vi "45-1523-1 State Diagram.vi"() -> ()   [LabVIEW 2015]
uses:
  Cases.ctl
  <vilib>/DAQmx/read.llb/DAQmx Read (Analog DBL 1Chan 1Samp).vi
  <vilib>/DAQmx/write.llb/DAQmx Write (Digital Bool 1Line 1Point).vi
  <vilib>/DAQmx/miscellaneous.llb/DAQmx Fill In Error Info.vi
  <vilib>/ErrorRing/Error Ring.xnode
  <vilib>/LabVIEW Interface for Arduino/LabVIEW Interface for Arduino.lvlib
panel:
  out "Numeric 3":dbl
  out "Numeric 2":dbl
  in  "EXIT Button":bool
  out "Numeric":dbl
  in  "Tab Control":T1(tab)
  in  "START Button":bool
  out "Slide":u8(slide) scale=0.0..100.0
  out "Slide 2":u8(slide) scale=0.0..100.0
  out "Slide 3":u8(slide) scale=0.0..100.0
  out "Slide 4":u8(slide) scale=0.0..100.0
  in  "Restart Button":bool
  in  "OK Button":bool
  in  "OK Button 10":bool
  in  "OK Button 3":bool
  in  "OK Button 4":bool
  in  "Restart Button 2":bool
  in  "START Button 2":bool caption="START Button"
  in  "OK Button 5":bool
  in  "OK Button 6":bool
  in  "OK Button 7":bool
  in  "OK Button 8":bool
  out "Slide 5":u8(slide) scale=0.0..100.0
  in  "OK Button 9":bool
  in  "OK Button 11":bool
  in  "OK Button 12":bool
  # "45-1523-1 Functional Tester"
  # "Click \"START TEST\" To Begin Test"
  # "TESTING J15..."
  # "TESTING K2..."
  # "TESTING K3..."
  # "TESTING K4..."
  # "ALL TESTS PASSED!"
  # "CHECK HIGHLIGHTED CONNECTIONS"
  # "SWITCH K2 FAILED!"
  # "SWITCH K3 FAILED!"
  # "SWITCH K4 FAILED!"
  # "Test Failed"
  # "Verify Connections, then Click \"START\""
  # "Possible Locations of Failure:\n   - Switch K1\n   - S1 Jumper\n   - Q4\n   - U1\n   - Q5"
  # "CHECK HIGHLIGHTED CONNECTIONS"
  # "Power Fault to Board"
  # "CHECK HIGHLIGHTED CONNECTION"
  # "TESTING DUT Power..."
  # "Are All Three LEDs Lit?"
  # "Possible Causes of Failure:\n   - LEDs (Reversed or Faulty)\n   - U1\n   - Q2"
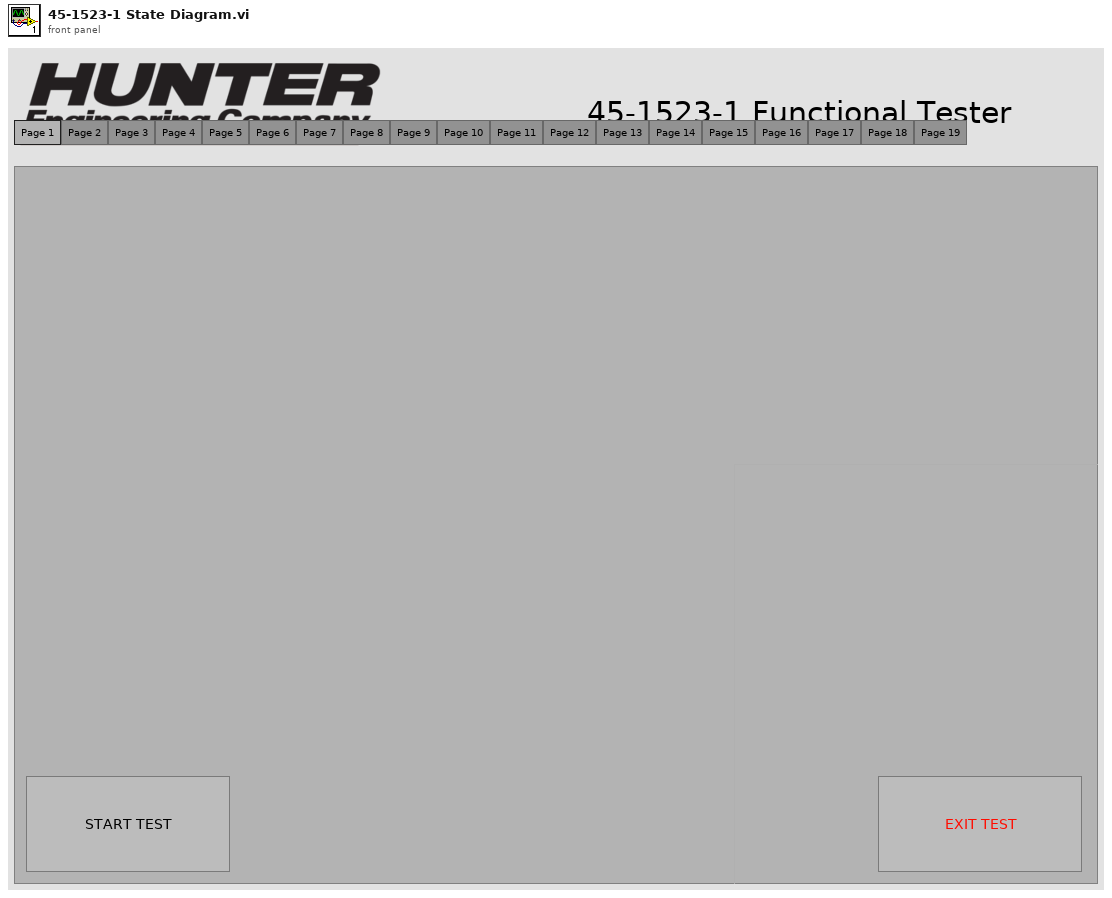
[diagram p1: front panel]
types:
  T1 = enum32{"Page 1", "Page 2", "Page 3", "Page 4", "Page 5", "Page 6", "Page 7", "Page 8", "Page 9", "Page 10", "Page 11", "Page 12", "Page 13", "Page 14", "Page 15", "Page 16", "Page 17", "Page 18", "Page 19"}
  T2 = typedef "Cases.ctl" = enum16{"Start", "Initalization", "J16 Test", "J15 Test", "J15 Error Page", "K2 Test", "K2 Error Page", "K3 Test", "K3 Error Page", "K4 Test", "K4 Error Page", "Test Complete", "Test Failed", "Error", "J15 Failed", "J16 Error", "J16 Failed", "K2 Failed", "LEDs Failed"}
  T3 = typedef "LabVIEW Interface for Arduino.lvlib/Arduino Resource.ctl" = cluster{"VISA resource":refnum<visa-resource-name>, "Board Type":T4, "Connection Type":enum8{"USB / Serial"}, "Bytes Per Packet (15)":u8}
  T4 = typedef "LabVIEW Interface for Arduino.lvlib/Board Type.ctl" = enum16{"Uno", "Dimuelanove w/Atmega 328", "Mega 2560"}
  T5 = enum8{"Enabled", "Disabled", "Disabled and Grayed Out"}
  T6 = enum32{"Page 1", "Page 2", "Page 3", "Page 4", "Page 5", "Page 6", "Page 7", "Page 8", "Page 9", "Page 10", "Page 11"}
  T7 = enum32{"Page 1", "Page 2", "Page 3", "Page 4", "Page 5", "Page 6", "Page 7", "Page 8", "Page 9", "Page 10", "Page 11", "Page 12"}
  T8 = enum32{"Page 1", "Page 2", "Page 3", "Page 4", "Page 5", "Page 6", "Page 7", "Page 8", "Page 9", "Page 10", "Page 11", "Page 12", "Page 13", "Page 14", "Page 15", "Page 16", "Page 17"}
  T9 = enum32{"Page 1", "Page 2", "Page 3", "Page 4", "Page 5", "Page 6", "Page 7", "Page 8", "Page 9", "Page 10", "Page 11", "Page 12", "Page 13", "Page 14", "Page 15", "Page 16", "Page 17", "Page 18"}
  T10 = enum32{"Page 1", "Page 2", "Page 3", "Page 4", "Page 5", "Page 6", "Page 7", "Page 8", "Page 9", "Page 10", "Page 11", "Page 12", "Page 13", "Page 14", "Page 15", "Page 16"}
  T11 = enum32{"Page 1", "Page 2", "Page 3", "Page 4", "Page 5", "Page 6", "Page 7", "Page 8", "Page 9", "Page 10", "Page 11", "Page 12", "Page 13"}
  T12 = enum32{"Page 1", "Page 2", "Page 3", "Page 4", "Page 5", "Page 6", "Page 7", "Page 8", "Page 9", "Page 10", "Page 11", "Page 12", "Page 13", "Page 14"}
  T13 = enum32{"Page 1", "Page 2", "Page 3", "Page 4", "Page 5", "Page 6", "Page 7", "Page 8", "Page 9", "Page 10", "Page 11", "Page 12", "Page 13", "Page 14", "Page 15"}
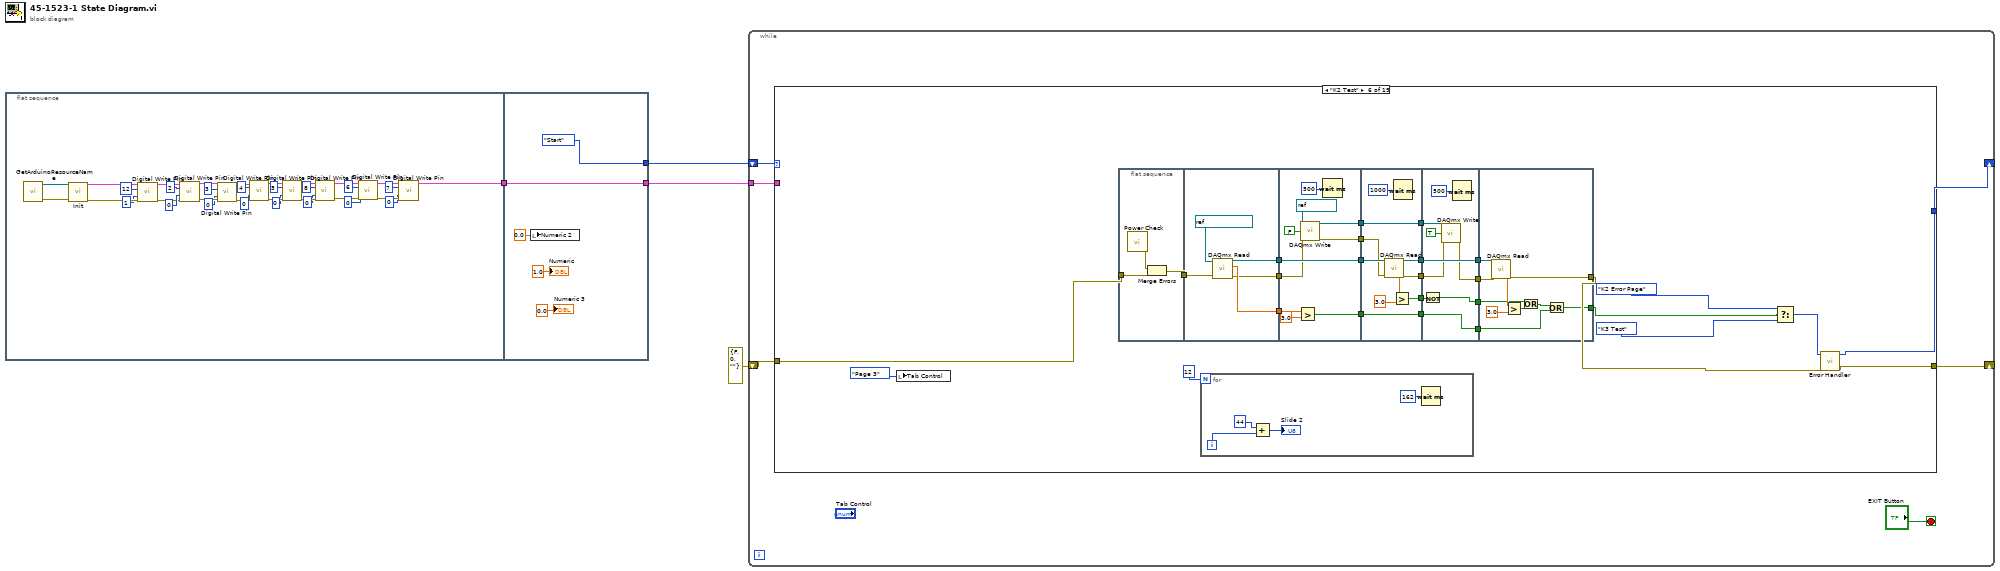
[diagram p0: block diagram]
diagram:
  n1 = flat-sequence {
    tunnel: [w11] -> w2
    tunnel: [Cases."Start" ("Enum")] -> w3
    tunnel: [w40] -> w1
    tunnel: w2 -> [w40]
    frame #0 {
      n2 = call "GetArduinoResourceName.vi"() -> ("error out"=w38:errorcluster, "VISA resource name"=w39:refnum<visa-resource-name>)  [unwired: 10 in]
      n3 = call <vilib>:"Init.vi"("VISA resource"=w39, "error in"=w38) -> ("Arduino Resource"=w10:T3, "error out"=w9:errorcluster)  [unwired: 16 in]
      n4 = call <vilib>:"Digital Write Pin.vi"("Arduino Resource"=w10, "Digital I/O Pin (0)"=u8 12, "Value (0)"=u8 1, "error in"=w9) -> ("Arduino Resource"=w7:T3, "error out"=w8:errorcluster)  [unwired: 10 in]
      n5 = call <vilib>:"Digital Write Pin.vi"("Arduino Resource"=w7, "Digital I/O Pin (0)"=u8 2, "Value (0)"=u8 0, "error in"=w8) -> ("Arduino Resource"=w37:T3, "error out"=w36:errorcluster)  [unwired: 10 in]
      n6 = call <vilib>:"Digital Write Pin.vi"("Arduino Resource"=w37, "Digital I/O Pin (0)"=u8 3, "Value (0)"=u8 0, "error in"=w36) -> ("Arduino Resource"=w35:T3, "error out"=w34:errorcluster)  [unwired: 10 in]
      n7 = call <vilib>:"Digital Write Pin.vi"("Arduino Resource"=w35, "Digital I/O Pin (0)"=u8 4, "Value (0)"=u8 0, "error in"=w34) -> ("Arduino Resource"=w33:T3, "error out"=w32:errorcluster)  [unwired: 10 in]
      n8 = call <vilib>:"Digital Write Pin.vi"("Arduino Resource"=w33, "Digital I/O Pin (0)"=u8 5, "Value (0)"=u8 0, "error in"=w32) -> ("Arduino Resource"=w31:T3, "error out"=w30:errorcluster)  [unwired: 10 in]
      n9 = call <vilib>:"Digital Write Pin.vi"("Arduino Resource"=w31, "Digital I/O Pin (0)"=u8 8, "Value (0)"=u8 0, "error in"=w30) -> ("Arduino Resource"=w19:T3, "error out"=w16:errorcluster)  [unwired: 10 in]
      n10 = call <vilib>:"Digital Write Pin.vi"("Arduino Resource"=w19, "Digital I/O Pin (0)"=u8 6, "Value (0)"=u8 0, "error in"=w16) -> ("Arduino Resource"=w14:T3, "error out"=w15:errorcluster)  [unwired: 10 in]
      n11 = call <vilib>:"Digital Write Pin.vi"("Arduino Resource"=w14, "Digital I/O Pin (0)"=u8 7, "Value (0)"=u8 0, "error in"=w15) -> ("Arduino Resource"=w11:T3)  [unwired: 10 in, 1 out]
    }
    frame #1 {
      n12 = local write "Numeric 2"(0.0 ("Numeric 2")) -> ()
      "Numeric" <- 1.0 ("Numeric")
      "Numeric 3" <- 0.0 ("Numeric 3")
    }
  }
  n13 = while {
    shift-right: [w49] -> _
    shift-left: w3 -> [w50]
    shift-right: [w47] -> _
    shift-left: errorcluster {"status"=FALSE, "code"=0, "source"=""} ("error out") -> [w46]
    tunnel: w1 -> [w45]
    stop <- "EXIT Button" stop-if-true
    n14 = case shown="\"K2 Test\"" w50 {
      tunnel: [w53 w78 w145 w206 w347 w383 w464 w479 w553 w575 w636 w645 w661 w680 w694 w706 w717 w727 w735] -> w49
      tunnel: [w55 w79 w144 w207 w348 w385 w465 w481 w556 w574 w635 w644 w660 w681 w693 w708 w719 w725 w737] -> w47
      tunnel: w46 -> [w51 w69 w142 w208 w342 w393 w466 w484 w555 w580 w634 w643 w653 w679 w692 w707 w720 w726 w736]
      tunnel: w45 -> [_ w68 w136 w177 w339 _ _ _ _ _ _ _ _ _ _ _ _ _ _]
      frame "Start" {
        n15 = property on="EXIT Button" class="Bool (strict)"("DisabledEnum"=T5."Enabled" ("Disabled")) -> ()  [unwired: 2 in, 2 out]
        n16 = while {
          stop <- w57 stop-if-true
          n17 = event shown="[0] \"START Button\", \"EXIT Button\": Value Change" {
            selector: _ -> [_]
            dyn-events: _ -> [_]
            timeout: _ -> [_]
            tunnel: ["START Button"] -> w57
            event "START Button", "EXIT Button": Value Change {
              n18 = event-data() -> ()  [unwired: 1 in, 6 out]
              n19 = local read "EXIT Button"() -> (w59:bool)
              n20 = case shown="False" w59 {
                tunnel: w59 -> [_ _]
                frame False {
                }
                frame True {
                  n21 = call "Shutdown VI.vi"() -> ()  [unwired: 12 in]
                }
              }
            }
          }
          n22 = local write "Tab Control"(T6."Page 1" ("Tab Control")) -> ()
        }
        n23 = call "Error Handler.vi"("error in (no error)"=w51, "Enum in"=Cases."Initalization") -> ("error out"=w55:errorcluster, "Enum out"=w53:T2)  [unwired: 8 in]
      }
      frame "Initalization", Default {
        n24 = local read "Numeric 2"() -> (w83:dbl)
        n25 = local write "Slide 5"(u8 0 ("Slide 5")) -> ()
        n26 = local write "Slide"(u8 22 ("Slide")) -> ()
        n27 = local write "Slide 2"(u8 40 ("Slide 2")) -> ()
        n28 = local write "Slide 3"(u8 52 ("Slide 3")) -> ()
        n29 = local write "Slide 4"(u8 67 ("Slide 4")) -> ()
        n30 = property on="EXIT Button" class="Bool (strict)"("DisabledEnum"=T5."Enabled" ("Disabled")) -> ()  [unwired: 2 in, 2 out]
        n31 = Equal?(x=2.0, y=w83) -> (x = y?=w82:bool)
        n32 = case shown="False" w82 {
          frame False {
          }
          frame True {
            "Numeric 2" <- 0.0 ("Numeric 2")
          }
        }
        n33 = flat-sequence {
          tunnel: [Cases."J16 Test" ("Enum")] -> w67
          tunnel: [w92] -> w65
          tunnel: w68 -> [w92]
          tunnel: w67 -> [w99]
          tunnel: [w99] -> w66
          tunnel: w65 -> [w98]
          tunnel: [w98] -> w64
          tunnel: w66 -> [w104]
          tunnel: [w104] -> w63
          tunnel: w64 -> [w103]
          tunnel: [w102] -> w61
          tunnel: w63 -> [w107]
          tunnel: [w107] -> w62
          tunnel: w61 -> [w106]
          tunnel: [w106] -> w60
          tunnel: w62 -> [w113]
          tunnel: [w114] -> w80
          tunnel: [w113] -> w77
          tunnel: w60 -> [w110]
          frame #0 {
            n34 = while {
              stop <- "START Button 2" stop-if-true
              n35 = local read "EXIT Button"() -> (w95:bool)
              n36 = case shown="False" w95 {
                frame False {
                }
                frame True {
                  n37 = call "Shutdown VI.vi"() -> ()  [unwired: 12 in]
                }
              }
            }
            n38 = local write "Tab Control"(T7."Page 12" ("Tab Control")) -> ()
          }
          frame #1 {
            n39 = Wait (ms)(milliseconds to wait=u32 1000) -> ()  [unwired: 1 out]
          }
          frame #2 {
            n40 = call <vilib>:"Digital Write Pin.vi"("Arduino Resource"=w103, "Digital I/O Pin (0)"=u8 8, "Value (0)"=u8 1) -> ("Arduino Resource"=w102:T3)  [unwired: 11 in, 1 out]
          }
          frame #3 {
            n41 = Wait (ms)(milliseconds to wait=u32 1000) -> ()  [unwired: 1 out]
          }
          frame #4 {
            n42 = call <vilib>:"Analog Read Pin.vi"("Arduino Resource"=w110, "Analog Input Pin (0)"=u8 1) -> ("Arduino Resource"=w108:T3, "Voltage"=w112:dbl, "error out"=w111:errorcluster)  [unwired: 11 in]
            n43 = Greater?(x=w112, y=3.0) -> (0:w116:bool)
            n44 = case shown="True" w116 {
              tunnel: [w118 w122] -> w115
              tunnel: w108 -> [_ w121]
              frame False {
                n45 = xnode "Error Ring"() -> ("error out"=w118:errorcluster)
              }
              frame True {
                n46 = flat-sequence {
                  tunnel: [w126] -> w123
                  tunnel: w121 -> [w128]
                  tunnel: [w124] -> w120
                  tunnel: [w131] -> w122
                  tunnel: w123 -> [w132]
                  tunnel: w120 -> [w130]
                  frame #0 {
                    n47 = call <vilib>:"Digital Write Pin.vi"("Arduino Resource"=w128, "Digital I/O Pin (0)"=u8 2, "Value (0)"=u8 0) -> ("Arduino Resource"=w124:T3, "error out"=w126:errorcluster)  [unwired: 11 in]
                    n48 = Wait (ms)(milliseconds to wait=u32 100) -> ()  [unwired: 1 out]
                  }
                  frame #1 {
                    (unwired) u8 1 ("Value (0)")
                    n49 = call <vilib>:"Digital Write Pin.vi"("Arduino Resource"=w130, "Digital I/O Pin (0)"=u8 2, "error in"=w132) -> ("error out"=w131:errorcluster)  [unwired: 11 in, 1 out]
                    n50 = Wait (ms)(milliseconds to wait=u32 100) -> ()  [unwired: 1 out]
                  }
                }
              }
            }
            n51 = Merge Errors(w115, w111) -> (w114:errorcluster)
          }
        }
        n52 = local read "Numeric"() -> (w74:dbl)
        n53 = Equal?(x=2.0, y=w74) -> (x = y?=w73:bool)
        n54 = case shown="False" w73 {
          frame False {
          }
          frame True {
            n55 = local write "Numeric"(0.0 ("Numeric")) -> ()
          }
        }
        n56 = local read "Numeric 3"() -> (w70:dbl)
        n57 = Equal?(x=2.0, y=w70) -> (x = y?=w72:bool)
        n58 = case shown="False" w72 {
          frame False {
          }
          frame True {
            n59 = local write "Numeric 3"(0.0 ("Numeric 3")) -> ()
          }
        }
        n60 = Merge Errors(w80, w69) -> (w84:errorcluster)
        n61 = call "Error Handler.vi"("error in (no error)"=w84, "Enum in"=w77) -> ("error out"=w79:errorcluster, "Enum out"=w78:T2)  [unwired: 8 in]
      }
      frame "J16 Test" {
        n62 = local write "Tab Control"(T8."Page 17" ("Tab Control")) -> ()
        n63 = property on="EXIT Button" class="Bool (strict)"("DisabledEnum"=T5."Disabled and Grayed Out" ("Disabled")) -> ()  [unwired: 2 in, 2 out]
        n64 = flat-sequence {
          tunnel: w142 -> [w155]
          tunnel: [w155] -> w140
          tunnel: [w156] -> w137
          tunnel: w136 -> [w156]
          tunnel: [w161] -> w149
          tunnel: w140 -> [w160]
          tunnel: w137 -> [w159]
          tunnel: w149 -> [w163]
          tunnel: [w162] -> w141
          tunnel: [w166] -> w148
          tunnel: w141 -> [w166]
          frame #0 {
            n65 = Wait (ms)(milliseconds to wait=u32 3000) -> ()  [unwired: 1 out]
          }
          frame #1 {
            n66 = call <vilib>:"Analog Read Pin.vi"("Arduino Resource"=w159, "Analog Input Pin (0)"=u8 6, "error in"=w160) -> ("Voltage"=w161:dbl)  [unwired: 10 in, 2 out]
          }
          frame #2 {
            n67 = Greater?(x=w163, y=2.5) -> (0:w162:bool)
            n68 = Wait (ms)(milliseconds to wait=u32 500) -> ()  [unwired: 1 out]
          }
          frame #3 {
          }
        }
        n69 = for {
          N: 22 -> [_]
          i -> [w153]
          n70 = Add(x=0, y=w153) -> (x+y=→"Slide 5":i32)
          n71 = Wait (ms)(milliseconds to wait=u32 162) -> ()  [unwired: 1 out]
        }
        n72 = Select(t=Cases."J16 Error" ("f"), s=w148, f=Cases."J15 Test") -> (s? t:f=w146:T2)
        n73 = call "Error Handler.vi"("Enum in"=w146) -> ("error out"=w144:errorcluster, "Enum out"=w145:T2)  [unwired: 9 in]
      }
      frame "J15 Test" {
        n74 = flat-sequence {
          tunnel: w208 -> [w283]
          tunnel: w177 -> [w280]
          tunnel: [w278] -> w176
          tunnel: [w277] -> w175
          tunnel: [w311] -> w211
          tunnel: w176 -> [w310]
          tunnel: w175 -> [w309]
          tunnel: [w306] -> w174
          tunnel: [w315] -> w212
          tunnel: w211 -> [w317]
          tunnel: [w318] -> w210
          tunnel: w174 -> [w316]
          tunnel: [w313] -> w173
          tunnel: w212 -> [w328]
          tunnel: w210 -> [w324]
          tunnel: [w325] -> w209
          tunnel: [w326] -> w204
          tunnel: w173 -> [w323]
          tunnel: [w320] -> w172
          tunnel: w209 -> [w335]
          tunnel: w204 -> [w336]
          tunnel: [w336] -> w201
          tunnel: [w334] -> w190
          tunnel: [w333] -> w181
          tunnel: w172 -> [w332]
          tunnel: [w330] -> w171
          frame #0 {
            n75 = call <vilib>:"Analog Read Pin.vi"("Arduino Resource"=w280) -> ("Arduino Resource"=w279:T3, "Voltage"=w281:dbl)  [unwired: 12 in, 1 out]
            n76 = Greater?(x=w281, y=3.0) -> (0:w285:bool)
            n77 = case shown="True" w285 {
              tunnel: [w286 w291] -> w284
              tunnel: w279 -> [_ w290]
              tunnel: [_ w288] -> w277
              frame False {
                n78 = xnode "Error Ring"() -> ("error out"=w286:errorcluster)
              }
              frame True {
                n79 = flat-sequence {
                  tunnel: [w297] -> w292
                  tunnel: w290 -> [w296]
                  tunnel: [w293] -> w289
                  tunnel: [w301] -> w291
                  tunnel: w292 -> [w302]
                  tunnel: w289 -> [w300]
                  tunnel: [w299] -> w288
                  frame #0 {
                    n80 = call <vilib>:"Digital Write Pin.vi"("Arduino Resource"=w296, "Digital I/O Pin (0)"=u8 2, "Value (0)"=u8 0) -> ("Arduino Resource"=w293:T3, "error out"=w297:errorcluster)  [unwired: 11 in]
                    n81 = Wait (ms)(milliseconds to wait=u32 100) -> ()  [unwired: 1 out]
                  }
                  frame #1 {
                    n82 = call <vilib>:"Digital Write Pin.vi"("Arduino Resource"=w300, "Digital I/O Pin (0)"=u8 2, "Value (0)"=u8 1, "error in"=w302) -> ("Arduino Resource"=w299:T3, "error out"=w301:errorcluster)  [unwired: 10 in]
                    n83 = Wait (ms)(milliseconds to wait=u32 100) -> ()  [unwired: 1 out]
                  }
                }
              }
            }
            n84 = Merge Errors(w284, w283) -> (w278:errorcluster)
          }
          frame #1 {
            n85 = call <vilib>:"Digital Write Pin.vi"("Arduino Resource"=w309, "Digital I/O Pin (0)"=u8 6, "Value (0)"=u8 0, "error in"=w310) -> ("Arduino Resource"=w306:T3, "error out"=w311:errorcluster)  [unwired: 10 in]
            n86 = Wait (ms)(milliseconds to wait=u32 500) -> ()  [unwired: 1 out]
          }
          frame #2 {
            n87 = call <vilib>:"Analog Read Pin.vi"("Arduino Resource"=w316, "Analog Input Pin (0)"=u8 1, "error in"=w317) -> ("Arduino Resource"=w313:T3, "Voltage"=w315:dbl, "error out"=w318:errorcluster)  [unwired: 10 in]
            n88 = Wait (ms)(milliseconds to wait=u32 500) -> ()  [unwired: 1 out]
          }
          frame #3 {
            n89 = Greater?(x=w328, y=3.0) -> (0:w326:bool)
            n90 = call <vilib>:"Digital Write Pin.vi"("Arduino Resource"=w323, "Digital I/O Pin (0)"=u8 2, "Value (0)"=u8 0, "error in"=w324) -> ("Arduino Resource"=w320:T3, "error out"=w325:errorcluster)  [unwired: 10 in]
            n91 = Wait (ms)(milliseconds to wait=u32 200) -> ()  [unwired: 1 out]
          }
          frame #4 {
            n92 = call <vilib>:"Analog Read Pin.vi"("Arduino Resource"=w332, "Analog Input Pin (0)"=u8 1, "error in"=w335) -> ("Arduino Resource"=w330:T3, "Voltage"=w333:dbl, "error out"=w334:errorcluster)  [unwired: 10 in]
            n93 = Wait (ms)(milliseconds to wait=u32 500) -> ()  [unwired: 1 out]
          }
        }
        n94 = local write "Tab Control"(T6."Page 2" ("Tab Control")) -> ()
        n95 = property on="EXIT Button" class="Bool (strict)"("DisabledEnum"=T5."Disabled and Grayed Out" ("Disabled")) -> ()  [unwired: 2 in, 2 out]
        n96 = for {
          N: 22 -> [_]
          i -> [w275]
          n97 = Add(x=22, y=w275) -> (x+y=→"Slide":i32)
          n98 = Wait (ms)(milliseconds to wait=u32 162) -> ()  [unwired: 1 out]
        }
        n99 = flat-sequence {
          tunnel: w181 -> [w218]
          tunnel: [w217] -> w180
          tunnel: [w215] -> w179
          tunnel: [w215] -> w178
          frame #0 {
            n100 = while {
              tunnel: ["OK Button 11"] -> w215
              stop <- w220 stop-if-true
              n101 = Or(x="OK Button 11", y="OK Button 9") -> (x .or. y?=w220:bool)
            }
            n102 = Greater?(x=w218, y=3.0) -> (0:w217:bool)
            n103 = local write "Tab Control"(T9."Page 18" ("Tab Control")) -> ()
          }
        }
        n104 = flat-sequence {
          tunnel: w180 -> [w232]
          tunnel: w201 -> [w231]
          tunnel: [w231] -> w197
          tunnel: [w230] -> w196
          tunnel: w190 -> [w228]
          tunnel: [w227] -> w189
          tunnel: w178 -> [w229]
          tunnel: w171 -> [w226]
          tunnel: [w223] -> w170
          tunnel: [w243] -> w198
          tunnel: w197 -> [w243]
          tunnel: w196 -> [w242]
          tunnel: [w242] -> w195
          tunnel: w189 -> [w241]
          tunnel: [w240] -> w188
          tunnel: w170 -> [w239]
          tunnel: [w236] -> w169
          tunnel: [w251] -> w199
          tunnel: w198 -> [w251]
          tunnel: w195 -> [w250]
          tunnel: [w250] -> w194
          tunnel: [w248] -> w191
          tunnel: w188 -> [w246]
          tunnel: w169 -> [w247]
          tunnel: [w245] -> w167
          tunnel: [w261] -> w200
          tunnel: w199 -> [w261]
          tunnel: w194 -> [w260]
          tunnel: [w260] -> w193
          tunnel: [w259] -> w192
          tunnel: w191 -> [w255]
          tunnel: [w256] -> w187
          tunnel: [w254] -> w168
          tunnel: w167 -> [w253]
          tunnel: w200 -> [w271]
          tunnel: w193 -> [w270]
          tunnel: w192 -> [w269]
          tunnel: w187 -> [w265]
          tunnel: [w266] -> w186
          tunnel: [w268] -> w182
          tunnel: w168 -> [w264]
          frame #0 {
            n105 = case shown="False" w229 {
              frame False {
                n106 = local write "Tab Control"(T9."Page 2" ("Tab Control")) -> ()
              }
              frame True {
                n107 = local write "Tab Control"(T1."Page 19" ("Tab Control")) -> ()
              }
            }
            n108 = Not(x=w232) -> (.not. x?=w230:bool)
            n109 = call <vilib>:"Digital Write Pin.vi"("Arduino Resource"=w226, "Digital I/O Pin (0)"=u8 6, "Value (0)"=u8 1, "error in"=w228) -> ("Arduino Resource"=w223:T3, "error out"=w227:errorcluster)  [unwired: 10 in]
            n110 = Wait (ms)(milliseconds to wait=u32 200) -> ()  [unwired: 1 out]
          }
          frame #1 {
            n111 = call <vilib>:"Digital Write Pin.vi"("Arduino Resource"=w239, "Digital I/O Pin (0)"=u8 7, "Value (0)"=u8 1, "error in"=w241) -> ("Arduino Resource"=w236:T3, "error out"=w240:errorcluster)  [unwired: 10 in]
            n112 = Wait (ms)(milliseconds to wait=u32 200) -> ()  [unwired: 1 out]
          }
          frame #2 {
            (unwired) u8 0 ("Value (0)")
            n113 = Wait (ms)(milliseconds to wait=u32 200) -> ()  [unwired: 1 out]
            n114 = call <vilib>:"Digital Write Pin.vi"("Arduino Resource"=w247, "Digital I/O Pin (0)"=u8 7, "error in"=w246) -> ("Arduino Resource"=w245:T3, "error out"=w248:errorcluster)  [unwired: 11 in]
          }
          frame #3 {
            n115 = call <vilib>:"Analog Read Pin.vi"("Arduino Resource"=w253, "Analog Input Pin (0)"=u8 1, "error in"=w255) -> ("Arduino Resource"=w254:T3, "Voltage"=w257:dbl, "error out"=w256:errorcluster)  [unwired: 10 in]
            n116 = Wait (ms)(milliseconds to wait=u32 500) -> ()  [unwired: 1 out]
            n117 = Greater?(x=w257, y=3.0) -> (0:w259:bool)
          }
          frame #4 {
            (unwired) u8 7 ("Digital I/O Pin (0)")
            n118 = Or(x=w270, y=w269) -> (x .or. y?=w272:bool)
            n119 = call <vilib>:"Digital Write Pin.vi"("Arduino Resource"=w264, "Value (0)"=u8 0, "error in"=w265) -> ("error out"=w266:errorcluster)  [unwired: 11 in, 1 out]
            n120 = Or(x=w271, y=w272) -> (x .or. y?=w268:bool)
          }
        }
        n121 = Select(t=Cases."J15 Error Page" ("Enum"), s=w182, f=Cases."K2 Test" ("Enum")) -> (s? t:f=w183:T2)
        n122 = Select(t=Cases."LEDs Failed" ("Enum"), s=w179, f=w183) -> (s? t:f=w203:T2)
        n123 = call "Error Handler.vi"("error in (no error)"=w186, "Enum in"=w203) -> ("error out"=w207:errorcluster, "Enum out"=w206:T2)  [unwired: 8 in]
      }
      frame "J15 Error Page" {
        n124 = call <vilib>:"Analog Read Pin.vi"("Arduino Resource"=w339, "error in"=w342) -> ("Arduino Resource"=w338:T3, "Voltage"=w340:dbl, "error out"=w341:errorcluster)  [unwired: 11 in]
        n125 = Greater?(x=w340, y=3.0) -> (0:w344:bool)
        n126 = case shown="True" w344 {
          tunnel: [w362 w366] -> w343
          tunnel: w338 -> [_ w365]
          frame False {
            n127 = xnode "Error Ring"() -> ("error out"=w362:errorcluster)
          }
          frame True {
            n128 = flat-sequence {
              tunnel: [w369] -> w367
              tunnel: w365 -> [w370]
              tunnel: [w368] -> w364
              tunnel: [w375] -> w366
              tunnel: w367 -> [w376]
              tunnel: w364 -> [w374]
              frame #0 {
                n129 = Wait (ms)(milliseconds to wait=u32 100) -> ()  [unwired: 1 out]
                n130 = call <vilib>:"Digital Write Pin.vi"("Arduino Resource"=w370, "Digital I/O Pin (0)"=u8 2, "Value (0)"=u8 0) -> ("Arduino Resource"=w368:T3, "error out"=w369:errorcluster)  [unwired: 11 in]
              }
              frame #1 {
                n131 = call <vilib>:"Digital Write Pin.vi"("Arduino Resource"=w374, "Digital I/O Pin (0)"=u8 2, "Value (0)"=u8 0, "error in"=w376) -> ("error out"=w375:errorcluster)  [unwired: 10 in, 1 out]
                n132 = Wait (ms)(milliseconds to wait=u32 100) -> ()  [unwired: 1 out]
              }
            }
          }
        }
        n133 = property on="EXIT Button" class="Bool (strict)"("DisabledEnum"=T5."Enabled" ("Disabled")) -> ()  [unwired: 2 in, 2 out]
        n134 = Merge Errors(w343, w341) -> ()  [unwired: 1 out]
        n135 = flat-sequence {
          tunnel: [w353] -> w346
          frame #0 {
            n136 = local read "Numeric"() -> (w350:dbl)
            n137 = Increment(x=w350) -> (x+1=w351:dbl)
            n138 = local write "Numeric"(w351) -> ()
          }
          frame #1 {
            n139 = local read "Numeric"() -> (w355:dbl)
            n140 = Quotient & Remainder(x=w355, y=2) -> (x-y*floor(x/y)=w354:dbl)  [unwired: 1 out]
            n141 = Equal To 0?(x=w354) -> (x = 0?=w352:bool)
            n142 = case shown="True" w352 {
              frame False {
              }
              frame True {
                n143 = local write "Tab Control"(T6."Page 7" ("Tab Control")) -> ()
              }
            }
            n144 = case shown="True" w352 {
              tunnel: [Cases."J15 Failed" ("Enum") Cases."Initalization" ("Enum")] -> w353
              frame False {
              }
              frame True {
                n145 = while {
                  stop <- "OK Button" stop-if-true
                  n146 = local read "EXIT Button"() -> (w360:bool)
                  n147 = case shown="True" w360 {
                    frame False {
                    }
                    frame True {
                      n148 = call "Shutdown VI.vi"() -> ()  [unwired: 12 in]
                    }
                  }
                }
              }
            }
          }
        }
        n149 = call "Error Handler.vi"("error in (no error)"=w341, "Enum in"=w346) -> ("error out"=w348:errorcluster, "Enum out"=w347:T2)  [unwired: 8 in]
      }
      frame "K2 Test" {
        n150 = local write "Tab Control"(T6."Page 3" ("Tab Control")) -> ()
        n151 = flat-sequence {
          tunnel: w393 -> [w413]
          tunnel: [w411] -> w381
          tunnel: [w417] -> w403
          tunnel: [w416] -> w399
          tunnel: [w414] -> w392
          tunnel: w381 -> [w415]
          tunnel: [w426] -> w406
          tunnel: w403 -> [w425]
          tunnel: [w425] -> w402
          tunnel: w399 -> [w424]
          tunnel: [w419] -> w394
          tunnel: w392 -> [w421]
          tunnel: [w420] -> w391
          tunnel: [w437] -> w405
          tunnel: w406 -> [w437]
          tunnel: w402 -> [w436]
          tunnel: [w435] -> w400
          tunnel: [w432] -> w398
          tunnel: [w431] -> w395
          tunnel: w394 -> [w431]
          tunnel: w391 -> [w430]
          tunnel: [w429] -> w390
          tunnel: w405 -> [w446]
          tunnel: [w444] -> w401
          tunnel: w400 -> [w444]
          tunnel: w398 -> [w443]
          tunnel: [w439] -> w397
          tunnel: [w442] -> w396
          tunnel: w395 -> [w442]
          tunnel: w390 -> [w441]
          tunnel: [w440] -> w389
          tunnel: [w453] -> w388
          tunnel: w401 -> [w457]
          tunnel: w397 -> [w454]
          tunnel: w396 -> [w451]
          tunnel: w389 -> [w450]
          tunnel: [w449] -> w380
          frame #0 {
            n152 = call "Power Check.vi"() -> ("error out"=w412:errorcluster)  [unwired: 11 in]
            n153 = Merge Errors(w412, w413) -> (w411:errorcluster)
          }
          frame #1 {
            n154 = call-poly <vilib>:"DAQmx Read.vi"("task/channels in"=refnum<k21> "Is K2 Closed", "error in"=w415) -> ("task out"=w417:refnum<k21>, "data"=w416:dbl, "error out"=w414:errorcluster)  [unwired: 11 in]
          }
          frame #2 {
            n155 = Greater?(x=w424, y=3.0) -> (0:w419:bool)
            n156 = call-poly <vilib>:"DAQmx Write.vi"("task/channels in"=refnum<k21> "Fire K2" ("DAQmx Task Name"), "data"=FALSE, "error in"=w421) -> ("task out"=w426:refnum<k21>, "error out"=w420:errorcluster)  [unwired: 10 in, 1 out]
            n157 = Wait (ms)(milliseconds to wait=u32 500) -> ()  [unwired: 1 out]
          }
          frame #3 {
            n158 = call-poly <vilib>:"DAQmx Read.vi"("task/channels in"=w436, "error in"=w430) -> ("task out"=w435:refnum<k21>, "data"=w433:dbl, "error out"=w429:errorcluster)  [unwired: 11 in]
            n159 = Greater?(x=w433, y=3.0) -> (0:w432:bool)
            n160 = Wait (ms)(milliseconds to wait=u32 1000) -> ()  [unwired: 1 out]
          }
          frame #4 {
            n161 = Not(x=w443) -> (.not. x?=w439:bool)
            n162 = call-poly <vilib>:"DAQmx Write.vi"("task/channels in"=w446, "data"=TRUE, "error in"=w441) -> ("error out"=w440:errorcluster)  [unwired: 10 in, 2 out]
            n163 = Wait (ms)(milliseconds to wait=u32 500) -> ()  [unwired: 1 out]
          }
          frame #5 {
            n164 = call-poly <vilib>:"DAQmx Read.vi"("task/channels in"=w457, "error in"=w450) -> ("data"=w455:dbl, "error out"=w449:errorcluster)  [unwired: 11 in, 1 out]
            n165 = Greater?(x=w455, y=3.0) -> (0:w448:bool)
            n166 = Or(x=w454, y=w448) -> (x .or. y?=w452:bool)
            n167 = Or(x=w452, y=w451) -> (x .or. y?=w453:bool)
          }
        }
        n168 = for {
          N: 12 -> [_]
          i -> [w409]
          n169 = Add(x=44, y=w409) -> (x+y=→"Slide 2":i32)
          n170 = Wait (ms)(milliseconds to wait=u32 162) -> ()  [unwired: 1 out]
        }
        n171 = Select(t=Cases."K2 Error Page" ("Enum"), s=w388, f=Cases."K3 Test" ("Enum")) -> (s? t:f=w384:T2)
        n172 = call "Error Handler.vi"("error in (no error)"=w380, "Enum in"=w384) -> ("error out"=w385:errorcluster, "Enum out"=w383:T2)  [unwired: 8 in]
      }
      frame "K2 Error Page" {
        n173 = while {
          stop <- TRUE stop-if-true
          n174 = local read "Numeric 3"() -> (w469:dbl)
          n175 = Increment(x=w469) -> (x+1=w468:dbl)
          n176 = local write "Numeric 3"(w468) -> ()
        }
        n177 = local write "Tab Control"(T10."Page 16" ("Tab Control")) -> ()
        n178 = property on="EXIT Button" class="Bool (strict)"("DisabledEnum"=T5."Enabled" ("Disabled")) -> ()  [unwired: 2 in, 2 out]
        n179 = local read "Numeric 3"() -> (w463:dbl)
        n180 = Quotient & Remainder(x=w463, y=2.0) -> (x-y*floor(x/y)=w461:dbl)  [unwired: 1 out]